vi "HFRR ADV v037.vi"() -> ()   [LabVIEW 2025] (continued)
                n805 = local write "EVENT LOG"(w838) -> ()
              }
            }
          }
        }
        n806 = case shown="True" w816 {
          frame False {
          }
          frame True {
            n807 = case shown="True" "Reach point temp" {
              selector: "Reach point temp" -> [_ w846]
              frame False {
              }
              frame True {
                n808 = local read "EVENT LOG"() -> (w843:string)
                n809 = Not(x=w846) -> (.not. x?=w845:bool)
                n810 = local write "Reach point temp"(w845) -> ()
                n811 = call "Event Log.vi"("Content"="Target Temperature reached", "EVENT LOG"=w843) -> ("EVENT LOG"=w844:string)  [unwired: 8 in, 1 out]
                n812 = local write "EVENT LOG"(w844) -> ()
              }
            }
          }
        }
        n813 = local read "Auto Start Test"() -> (w819:bool)
        n814 = And(x=w816, y=w815) -> (x .and. y?=w825:bool)
        n815 = Select(t=Auto_Start_enum."Maintain Stage" ("Enum - Selector"), s=w825, f=Auto_Start_enum."Reach point" ("Enum - Selector")) -> (s? t:f=w822:T15)
        n816 = Not(x=w819) -> (.not. x?=w818:bool)
        n817 = Select(t=Auto_Start_enum."close", s=w818, f=w822) -> (s? t:f=w820:T15)
        n818 = call "ELAPSED TIMER VI.vi"("RESET"=w821, "PAUSE"=w821) -> ()  [unwired: 7 in, 3 out]
      }
      frame "Maintain Stage" {
        w861 = 2.0 ("y")
        w860 = 1.0 ("y")
        # "Humidity and  temperatures Set Point  have been reached"
        n819 = local read "Set Temp"() -> (w847:dbl)
        n820 = local read "Set Humidity:"() -> (w864:dbl)
        n821 = local read "Humidity ( %RH )"() -> (w867:dbl)
        n822 = Add(x=w847, y=w860) -> (x+y=w866:dbl)
        n823 = Subtract(x=w847, y=w860) -> (x-y=w865:dbl)
        n824 = local read "TEMP"() -> (w868:dbl)
        n825 = Add(x=w864, y=w861) -> (x+y=w863:dbl)
        n826 = Subtract(x=w864, y=w861) -> (x-y=w862:dbl)
        n827 = In Range and Coerce(upper limit=w866, x=w868, lower limit=w865) -> (In Range?=w859:bool)  [unwired: 1 out]
        n828 = In Range and Coerce(upper limit=w863, x=w867, lower limit=w862) -> (In Range?=w858:bool)  [unwired: 1 out]
        n829 = And(x=w859, y=w858) -> (x .and. y?=w857:bool)
        n830 = Not(x=w857) -> (.not. x?=w856:bool)
        n831 = call "ELAPSED TIMER VI.vi"("TARGET"=60.0, "RESET"=w856, "PAUSE"=FALSE) -> ("ELAPSED INDICATION"=w853:bool)  [unwired: 6 in, 2 out]
        n832 = case shown="True" w853 {
          tunnel: w853 -> [_ w871]
          tunnel: [Auto_Start_enum."Maintain Stage" ("Enum - Selector") w870] -> w851
          frame False {
          }
          frame True {
            n833 = stacked-sequence {
              tunnel: w871 -> [_ _ _ _ _]
              tunnel: [_ _ _ _ Auto_Start_enum."Start Stage" ("Enum - Selector")] -> w870
              frame #0 {
                n834 = local read "EVENT LOG"() -> (w873:string)
                n835 = call "Event Log.vi"("Content"="Humidity and temperature set point has stabilized.", "EVENT LOG"=w873) -> ("EVENT LOG"=w874:string)  [unwired: 8 in, 1 out]
                n836 = local write "EVENT LOG"(w874) -> ()
              }
              frame #1 {
                n837 = Wait (ms)(milliseconds to wait=u32 100) -> ()  [unwired: 1 out]
              }
              frame #2 {
                n838 = local read "EVENT LOG"() -> (w877:string)
                n839 = call "Event Log.vi"("Content"="Auto Test Started", "EVENT LOG"=w877) -> ("EVENT LOG"=w878:string)  [unwired: 8 in, 1 out]
                n840 = local write "EVENT LOG"(w878) -> ()
              }
              frame #3 {
                w879 = TRUE ("RUN")
                n841 = local write "RUN"(w879) -> ()
                n842 = property on="Auto Start Temp" class="Bool (strict)"("Val(Sgnl)"=w879) -> ()  [unwired: 2 in, 2 out]
                "Auto Start Temp" <- w879
              }
              frame #4 {
              }
            }
          }
        }
        n843 = local read "Auto Start Test"() -> (w850:bool)
        n844 = Not(x=w850) -> (.not. x?=w849:bool)
        n845 = Select(t=Auto_Start_enum."close", s=w849, f=w851) -> (s? t:f=w852:T15)
      }
      frame "Start Stage" {
        w881 = TRUE ("PAUSE")
        n846 = local read "Auto Start Test"() -> (w886:bool)
        n847 = Not(x=w886) -> (.not. x?=w885:bool)
        n848 = Select(t=Auto_Start_enum."close" ("Enum - Selector"), s=w885, f=Auto_Start_enum."Start Stage" ("Enum - Selector")) -> (s? t:f=w882:T15)
        n849 = call "ELAPSED TIMER VI.vi"("RESET"=w881, "PAUSE"=w881) -> ()  [unwired: 7 in, 3 out]
      }
      frame "close" {
        w889 = FALSE ("Heater Button")
        n850 = local write "RUN"(w889) -> ()
        n851 = local write "Heater Button"(w889) -> ()
        n852 = local write "Humidity"(w889) -> ()
        n853 = local write "Auto Start Test"(w889) -> ()
        n854 = property on="Heater Button" class="Bool (strict)"("Val(Sgnl)"=FALSE ("Value (Signaling)")) -> ()  [unwired: 2 in, 2 out]
        n855 = local write "Humidity"(TRUE ("Humidity")) -> ()
      }
      frame "Exit" {
      }
    }
    n856 = Wait (ms)(milliseconds to wait=u32 100) -> ()  [unwired: 1 out]
    n857 = local read "Quit"() -> (w784:bool)
  }
  n858 = property on="Service Password Log" class="Str"("Visible"=w21) -> ()  [unwired: 2 in, 2 out]
  n859 = property on="Password 3" class="Clust (strict)"("Visible"=w21) -> ()  [unwired: 2 in, 2 out]
  n860 = while {
    stop <- w918 stop-if-true
    w901 = errorcluster {"status"=FALSE, "code"=0, "source"=""} ("error in (no error) 3")
    # "this loop is for manual report generation"
    n861 = local read "Confirm Measrurement"() -> (w900:bool)
    n862 = case shown="True" w900 {
      selector: w900 -> [_ w1008]
      tunnel: errorcluster {"status"=FALSE, "code"=0, "source"=""} ("error in (no error) 3") -> [_ w1009]
      tunnel: [_ w1007] -> _
      frame False {
      }
      frame True {
        n863 = stacked-sequence {
          tunnel: w1009 -> [_ w1042 _]
          tunnel: w1008 -> [_ _ w1149]
          tunnel: [_ w1030 _] -> w1007
          frame #0 {
            n864 = String To Path(string="C:\\LAB-IQ\\Image Calibrate v01.dcf") -> (path=w1012:path)
            n865 = Open/Create/Replace File ("Open File")(file path (use dialog)=w1012) -> (refnum out=w1013:refnum<file>)  [unwired: 5 in, 2 out]
            n866 = for {
              N: 4 -> [_]
              tunnel: w1013 -> [w1019]
              i -> [w1015]
              n867 = Read from Text File ("Read File")(file (use dialog)=w1019) -> (text=w1020:string)  [unwired: 3 in, 3 out]
              n868 = String Subset(string=w1020, offset (0)=6, length (rest)=10 ("length (rest)")) -> (substring=w1016:string)
              n869 = Fract/Exp String To Number(string=w1016) -> (number=w1014:dbl)  [unwired: 3 in, 1 out]
              n870 = case shown="3" w1015 {
                tunnel: w1014 -> [w1021 w1022 _ w1023 _]
                frame 0 {
                  n871 = local write "5x Gain"(w1021) -> ()
                }
                frame 1 {
                  n872 = local write "10x Gain"(w1022) -> ()
                }
                frame 2 {
                }
                frame 3 {
                  n873 = local write "100x gain"(w1023) -> ()
                }
                frame 4, Default {
                }
              }
            }
          }
          frame #1 {
            n874 = local read "TEST STANDARD"() -> (w1025:T3)
            n875 = case shown="\"ISO 12156\"" w1025 {
              tunnel: ["ASTM D6079" "ISO 12156"] -> w1024
              frame "ASTM D6079", Default {
              }
              frame "ISO 12156" {
              }
            }
            n876 = call "IMAGE ANALYSIS.vi"("Enum"=POST_ANALYSIS_ENUM."GET MEASUREMENTS", "error in"=w1042) -> ("error out"=w1049:errorcluster)  [unwired: 8 in, 1 out]
            n877 = local read "Magnification :"() -> (w1035:string)
            n878 = call "Stall Data Flow.vim"("value in"=w1049, "milliseconds to wait"=u32 1000) -> ("value out"=w1048:errorcluster)  [unwired: 1 out]
            n879 = local read "Test File List :"() -> (w1046:string)
            n880 = case shown="\"10x\"" w1035 {
              tunnel: [w1085 w1086] -> w1033
              frame "5x", Default {
                n881 = local read "5x Gain"() -> (w1085:dbl)
              }
              frame "10x" {
                # "5x"
                n882 = local read "10x Gain"() -> (w1086:dbl)
              }
            }
            n883 = call "IMAGE ANALYSIS.vi"("Enum"=POST_ANALYSIS_ENUM."READ", "error in"=w1048) -> ("error out"=w1045:errorcluster, "data out"=w1036:string)  [unwired: 8 in]
            n884 = Match Pattern(string=w1036, regular expression="\"type\": ") -> (after substring=w1040:string)  [unwired: 1 in, 3 out]
            n885 = call "IMAGE PATH CREATION PY.vi"("error in (no error)"=w1045, "File Name :"=w1046) -> ("error out"=w1044:errorcluster, "File Path"=w1032:path, "File Path String:"=w1027:string)  [unwired: 7 in]
            n886 = Match Pattern(string=w1040, regular expression=",") -> (before substring=w1026:string)  [unwired: 1 in, 3 out]
            n887 = local read "Calibration Tab"() -> (w1029:enum32{"Measrument", "Calibrate"})
            n888 = call "Stall Data Flow.vim"("value in"=w1044, "milliseconds to wait"=u32 250) -> ("value out"=w1028:errorcluster)  [unwired: 1 out]
            n889 = Equal?(x=w1026, y="\"rectangle\"") -> (x = y?=w1037:bool)
            n890 = case shown="False" w1037 {
              tunnel: w1036 -> [w1091 w1146]
              tunnel: w1033 -> [_ w1137]
              tunnel: cluster{"major":dbl, "minor":dbl, "average":dbl} {"major"=0.0, "minor"=0.0, "average"=0.0} -> [w1089 w1133]
              tunnel: [w1088 w1130] -> w1031
              tunnel: w1026 -> [w1090 _]
              tunnel: w1033 -> [w1087 _]
              frame False {
                n891 = Equal?(x=w1090, y="\"line\"") -> (x = y?=w1092:bool)
                n892 = case shown="True" w1092 {
                  tunnel: w1091 -> [_ w1107]
                  tunnel: w1089 -> [w1094 w1106]
                  tunnel: [w1094 w1104] -> w1088
                  tunnel: w1087 -> [_ w1103]
                  frame False {
                  }
                  frame True {
                    w1102 = 0.0 ("Major Axis")
                    n893 = Match Pattern(string=w1107, regular expression="\"length_px\":") -> (after substring=w1105:string)  [unwired: 1 in, 3 out]
                    n894 = property on="Major Axis" class="DigNum (strict)"("Caption.Text"="") -> ()  [unwired: 2 in, 2 out]
                    n895 = property on="Minor Axis" class="DigNum (strict)"("Caption.Text"="") -> ()  [unwired: 2 in, 2 out]
                    n896 = property on="Average" class="DigNum (strict)"("Caption.Text"="Line") -> ()  [unwired: 2 in, 2 out]
                    n897 = Fract/Exp String To Number(string=w1105, default (0 dbl)=0.0 ("default (0 DBL)")) -> (number=w1101:dbl)  [unwired: 2 in, 1 out]
                    "Pixel Value" <- w1101
                    n898 = Multiply(x=w1101, y=w1103) -> (x*y=w1114:dbl)
                    n899 = Multiply(x=w1114, y=1000.0) -> (x*y=w1097:dbl)
                    n900 = Divide(x=w1097, y=1000.0) -> (x/y=w1100:dbl)
                    n901 = local write "Measurment (mm)"(w1100) -> ()
                    n902 = Bundle By Name(cluster=w1106, "average"=w1097) -> (w1104:cluster{"major":dbl, "minor":dbl, "average":dbl})
                    n903 = Number To Fractional String(number=w1097, precision (6)=i16 1) -> (F-format string=w1096:string)  [unwired: 2 in]
                    n904 = local write "Minor Axis"(w1102) -> ()
                    n905 = local write "Major Axis"(w1102) -> ()
                    n906 = Fract/Exp String To Number(string=w1096) -> (number=w1095:dbl)  [unwired: 3 in, 1 out]
                    n907 = local write "Average"(w1095) -> ()
                  }
                }
              }
              frame True {
                w1134 = 1000.0 ("y")
                w1140 = 0.0 ("default (0 DBL)")
                n908 = Match Pattern(string=w1146, regular expression=" \"width_px\":") -> (after substring=w1144:string)  [unwired: 1 in, 3 out]
                n909 = Match Pattern(string=w1144, regular expression="\"height_px\":") -> (before substring=w1142:string, after substring=w1141:string)  [unwired: 1 in, 2 out]
                n910 = Fract/Exp String To Number(string=w1142, default (0 dbl)=w1140) -> (number=w1139:dbl)  [unwired: 2 in, 1 out]
                n911 = Fract/Exp String To Number(string=w1141, default (0 dbl)=w1140) -> (number=w1138:dbl)  [unwired: 2 in, 1 out]
                n912 = Multiply(x=w1139, y=w1137) -> (x*y=w1136:dbl)
                n913 = Multiply(x=w1138, y=w1137) -> (x*y=w1135:dbl)
                n914 = Multiply(x=w1136, y=w1134) -> (x*y=w1120:dbl)
                n915 = Multiply(x=w1135, y=w1134) -> (x*y=w1118:dbl)
                n916 = Add(x=w1120, y=w1118) -> (x+y=w1132:dbl)
                n917 = property on="Major Axis" class="DigNum (strict)"("Caption.Text"="Major Axis") -> ()  [unwired: 2 in, 2 out]
                n918 = property on="Minor Axis" class="DigNum (strict)"("Caption.Text"="Minor Axis") -> ()  [unwired: 2 in, 2 out]
                n919 = property on="Average" class="DigNum (strict)"("Caption.Text"="Average") -> ()  [unwired: 2 in, 2 out]
                n920 = Divide(x=w1132, y=2.0) -> (x/y=w1116:dbl)
                n921 = Bundle By Name(cluster=w1133, "major"=w1120, "minor"=w1118, "average"=w1116) -> (w1130:cluster{"major":dbl, "minor":dbl, "average":dbl})
                n922 = Number To Fractional String(number=w1118, precision (6)=i16 1) -> (F-format string=w1125:string)  [unwired: 2 in]
                n923 = Number To Fractional String(number=w1116, precision (6)=i16 1) -> (F-format string=w1126:string)  [unwired: 2 in]
                n924 = Number To Fractional String(number=w1120, precision (6)=i16 1) -> (F-format string=w1124:string)  [unwired: 2 in]
                n925 = Fract/Exp String To Number(string=w1125) -> (number=w1117:dbl)  [unwired: 3 in, 1 out]
                n926 = Fract/Exp String To Number(string=w1126) -> (number=w1115:dbl)  [unwired: 3 in, 1 out]
                n927 = Fract/Exp String To Number(string=w1124) -> (number=w1119:dbl)  [unwired: 3 in, 1 out]
                n928 = local write "Major Axis"(w1119) -> ()
                n929 = local write "Average"(w1115) -> ()
                n930 = local write "Minor Axis"(w1117) -> ()
              }
            }
            n931 = case shown="\"Measrument\", Default" w1029 {
              tunnel: w1032 -> [w1059 _]
              tunnel: w1031 -> [w1058 _]
              tunnel: [w1055 w1084] -> w1030
              tunnel: w1028 -> [w1057 w1084]
              tunnel: w1027 -> [w1056 _]
              tunnel: w1024 -> [w1054 _]
              frame "Measrument", Default {
                n932 = stacked-sequence {
                  tunnel: w1059 -> [w1077 _]
                  tunnel: w1058 -> [w1075 _]
                  tunnel: w1057 -> [w1073 _]
                  tunnel: w1056 -> [w1072 _]
                  tunnel: [w1067 _] -> w1055
                  tunnel: w1054 -> [w1060 _]
                  frame #0 {
                    n933 = call "IMAGE ANALYSIS.vi"("Enum"=POST_ANALYSIS_ENUM."SAVE IMAGE", "error in"=w1073, "IMAGE FILE PATH"=w1072) -> ("error out"=w1071:errorcluster)  [unwired: 7 in, 1 out]
                    n934 = call "Stall Data Flow.vim"("value in"=w1071, "milliseconds to wait"=u32 1000) -> ("value out"=w1062:errorcluster)  [unwired: 1 out]
                    n935 = local read "Test File List :"() -> (w1079:string)
                    n936 = call "IMAGE ANALYSIS.vi"("Enum"=POST_ANALYSIS_ENUM."MINIMIZE UI", "error in"=w1062) -> ("error out"=w1069:errorcluster)  [unwired: 8 in, 1 out]
                    n937 = Bundle By Name(cluster=T27 {"File Name"="", "Test Method"="", "Operator"="", "Fuel Description"="", "Date and time"=""} ("Main Ref"), "Test Method"=w1060, "File Name"=w1079) -> (w1080:T27)
                    n938 = call "Stall Data Flow.vim"("value in"=w1069, "milliseconds to wait"=u32 1500) -> ("value out"=w1064:errorcluster)  [unwired: 1 out]
                    n939 = call "duf file read.vi"("error in (no error)"=w1064, "Main Ref"=w1080) -> ("error out"=w1078:errorcluster, "Main Ref 2"=w1076:T27)  [unwired: 8 in]
                    n940 = call "DETECTION REPORT for manual.vi"("error in (no error)"=w1078, "return value 3"=w1075, "Image File Path"=w1077, "Main Ref"=w1076) -> ("error out"=w1074:errorcluster)  [unwired: 7 in]
                    n941 = call <vilib>:"Clear Errors.vi"("error in (no error)"=w1074) -> ("error out"=w1065:errorcluster)  [unwired: 5 in, 1 out]
                    n942 = call "IMAGE ANALYSIS.vi"("Enum"=POST_ANALYSIS_ENUM."MINIMIZE UI", "error in"=w1065) -> ("error out"=w1067:errorcluster)  [unwired: 8 in, 1 out]
                  }
                  frame #1 {
                    n943 = local write "Main Tab"(T2."HOME" ("Main Tab")) -> ()
                    n944 = local write "Main Dashboard Buttons"(T1."Home" ("Main Dashboard Buttons")) -> ()
                  }
                }
              }
              frame "Calibrate" {
              }
            }
          }
          frame #2 {
            n945 = Not(x=w1149) -> (.not. x?=w1148:bool)
            n946 = local write "Confirm Measrurement"(w1148) -> ()
            n947 = local read "Calibration Tab"() -> (w1147:enum32{"Measrument", "Calibrate"})
            n948 = case shown="\"Measrument\", Default" w1147 {
              frame "Measrument", Default {
                (unwired) T21."HOME" ("Main Tab")
                n949 = local write "Main Tab"(T2."HOME" ("Main Tab")) -> ()
              }
              frame "Calibrate" {
              }
            }
          }
        }
      }
    }
    n950 = local read "Humidity"() -> (w892:bool)
    n951 = local read "Save Change"() -> (w897:bool)
    n952 = local read "Calibrate"() -> (w898:bool)
    n953 = local read "Auto Start Test"() -> (w893:bool)
    n954 = case shown="True" w898 {
      selector: w898 -> [_ w1005]
      frame False {
      }
      frame True {
        n955 = Not(x=w1005) -> (.not. x?=w1004:bool)
        n956 = local write "Calibrate"(w1004) -> ()
        n957 = local write "Calibration Tab"(enum32{"Measrument", "Calibrate"}."Calibrate" ("Calibration Tab")) -> ()
      }
    }
    n958 = case shown="True" w897 {
      selector: w897 -> [_ w949]
      frame False {
      }
      frame True {
        n959 = stacked-sequence {
          tunnel: w949 -> [_ _ _ _ w1003]
          frame #0 {
            n960 = call "IMAGE ANALYSIS.vi"("Enum"=POST_ANALYSIS_ENUM."HIDE UI") -> ()  [unwired: 9 in, 2 out]
          }
          frame #1 {
            n961 = local read "100x gain"() -> (w951:dbl)
            n962 = local read "10x Gain"() -> (w952:dbl)
            n963 = local read "5x Gain"() -> (w953:dbl)
            n964 = Number To Fractional String(number=w952, width (-)=i16 4, precision (6)=i16 7) -> (F-format string=w974:string)  [unwired: 1 in]
            n965 = Number To Fractional String(number=0.0, width (-)=i16 4, precision (6)=i16 7) -> (F-format string=w969:string)  [unwired: 1 in]
            n966 = Number To Fractional String(number=w951, width (-)=i16 4, precision (6)=i16 7) -> (F-format string=w957:string)  [unwired: 1 in]
            n967 = Number To Fractional String(number=w953, width (-)=i16 10 ("precision (6)"), precision (6)=i16 7) -> (F-format string=w983:string)  [unwired: 1 in]
            n968 = Concatenate Strings("[CH1]" ("string"), w983, " - 5x Gain" ("string"), "\r") -> (w973:string)
            n969 = Concatenate Strings("[CH2]" ("string"), w974, " - 10x Gain" ("string"), "\r") -> (w972:string)
            n970 = Concatenate Strings("[CH3]" ("string"), w969, " - 20x Gain" ("string"), "\r") -> (w963:string)
            n971 = Concatenate Strings("[CH4]" ("string"), w957, " - 100x Gain" ("string"), "\r") -> (w956:string)
            n972 = String To Path(string="C:\\LAB-IQ\\Image Calibrate v01.dcf") -> (path=w986:path)
            n973 = Concatenate Strings(w973, w972, w963, w956) -> (w971:string)
            n974 = call <vilib>:"Write Characters To File.vi"("append to file? (new file:F)"=FALSE, "character string"=w971, "file path (dialog if empty)"=w986) -> ()  [unwired: 2 in, 1 out]
          }
          frame #2 {
            n975 = String To Path(string="C:\\LAB-IQ\\Image Calibrate v01.dcf") -> (path=w989:path)
            n976 = Open/Create/Replace File ("Open File")(file path (use dialog)=w989) -> (refnum out=w990:refnum<file>)  [unwired: 5 in, 2 out]
            n977 = for {
              N: 4 -> [_]
              tunnel: w990 -> [w996]
              i -> [w992]
              n978 = Read from Text File ("Read File")(file (use dialog)=w996) -> (text=w997:string)  [unwired: 3 in, 3 out]
              n979 = String Subset(string=w997, offset (0)=6, length (rest)=10 ("length (rest)")) -> (substring=w993:string)
              n980 = Fract/Exp String To Number(string=w993) -> (number=w991:dbl)  [unwired: 3 in, 1 out]
              n981 = case shown="3" w992 {
                tunnel: w991 -> [w998 w999 _ w1000 _]
                frame 0 {
                  n982 = local write "5x Gain"(w998) -> ()
                }
                frame 1 {
                  n983 = local write "10x Gain"(w999) -> ()
                }
                frame 2 {
                }
                frame 3 {
                  n984 = local write "100x gain"(w1000) -> ()
                }
                frame 4, Default {
                }
              }
            }
          }
          frame #3 {
            n985 = call "IMAGE ANALYSIS.vi"("Enum"=POST_ANALYSIS_ENUM."SHOW UI") -> ()  [unwired: 9 in, 2 out]
          }
          frame #4 {
            n986 = Not(x=w1003) -> (.not. x?=w1002:bool)
            n987 = local write "Save Change"(w1002) -> ()
          }
        }
      }
    }
    n988 = case shown="False" w893 {
      tunnel: w892 -> [w919 _]
      frame False {
        n989 = case shown="True" w919 {
          frame False {
          }
          frame True {
            n990 = local read "Set Humidity:"() -> (w923:dbl)
            n991 = local read "Set Humidity:"() -> (w926:dbl)
            n992 = local read "Humidity ( %RH )"() -> (w927:dbl)
            n993 = Subtract(x=w923, y=2.0) -> (x-y=w921:dbl)
            n994 = Add(x=w926, y=2.0) -> (x+y=w922:dbl)
            n995 = In Range and Coerce(upper limit=w922, x=w927, lower limit=w921) -> (In Range?=w920:bool)  [unwired: 1 out]
            n996 = case shown="True" w920 {
              frame False {
              }
              frame True {
                n997 = case shown="True" "Manual Humididty Reached" {
                  selector: "Manual Humididty Reached" -> [_ w930]
                  frame False {
                  }
                  frame True {
                    n998 = Not(x=w930) -> (.not. x?=w929:bool)
                    n999 = local write "Manual Humididty Reached"(w929) -> ()
                    n1000 = local read "EVENT LOG"() -> (w932:string)
                    n1001 = call "Event Log.vi"("Content"="Target Humidity reached", "EVENT LOG"=w932) -> ("EVENT LOG"=w931:string)  [unwired: 8 in, 1 out]
                    n1002 = local write "EVENT LOG"(w931) -> ()
                  }
                }
              }
            }
          }
        }
      }
      frame True {
        n1003 = local write "Manual Humididty Reached"(TRUE ("Manual Humididty Reached")) -> ()
      }
    }
    n1004 = local read "Cap Live Image"() -> (w913:bool)
    n1005 = local read "SCAR MEASURMENT"() -> (w916:enum32{"Auto Scar", "Manual Scar"})
    n1006 = Wait (ms)(milliseconds to wait=u32 250) -> ()  [unwired: 1 out]
    n1007 = Equal?(x=w916, y=enum32{"Auto Scar", "Manual Scar"}."Manual Scar" ("SCAR MEASURMENT")) -> (x = y?=w914:bool)
    n1008 = And(x=w914, y=w913) -> (x .and. y?=w912:bool)
    n1009 = case shown="True" w912 {
      selector: w912 -> [_ w1228]
      frame False {
      }
      frame True {
        n1010 = stacked-sequence {
          tunnel: [_ _ _ w1243 _] -> _
          tunnel: w1228 -> [_ _ _ _ w1250]
          frame #0 {
            w1229 = 0.0
            n1011 = local write "Major Axis"(w1229) -> ()
            n1012 = local write "Minor Axis"(w1229) -> ()
            n1013 = local write "Average"(w1229) -> ()
          }
          frame #1 {
            n1014 = call "CAMERA LIVE FEED FGV.vi"("Enum - Menu"=CAMERA_LIVE_FEED_ENUM."CAMERA MINIMIZE") -> ()  [unwired: 9 in, 2 out]
          }
          frame #2 {
            n1015 = local read "FILE 3"() -> (w1237:string)
            n1016 = call <vilib>:"Trim Whitespace.vi"("string"="C:\\LAB-IQ\\images\\") -> ("trimmed string"=w1239:string)  [unwired: 1 in]
            n1017 = String To Path(string=w1239) -> (path=w1238:path)
            n1018 = Concatenate Strings(w1237, ".png" ("string")) -> (w1236:string)
            n1019 = Build Path(base path=w1238, name or relative path=w1236) -> (appended path=w1234:path)
            n1020 = Path To String(path=w1234) -> (string=w1233:string)
            n1021 = call "CAMERA LIVE FEED FGV.vi"("Enum - Menu"=CAMERA_LIVE_FEED_ENUM."CAMERA SAVE", "Image Path"=w1233) -> ("error out"=w1231:errorcluster)  [unwired: 8 in, 1 out]
            n1022 = case shown="No Error" w1231 {
              frame No Error {
                n1023 = One Button Dialog(message="Image saved successfully") -> ()  [unwired: 1 in, 1 out]
              }
              frame Error {
              }
            }
          }
          frame #3 {
            n1024 = call "LIST FILE NAMES.vi"() -> ("error out"=w1245:errorcluster, "filenames"=w1242:string[])  [unwired: 10 in]
            n1025 = call "IMAGE ANALYSIS.vi"("Enum"=POST_ANALYSIS_ENUM."SHOW UI", "error in"=w1245) -> ("error out"=w1243:errorcluster)  [unwired: 8 in, 1 out]
            n1026 = property on="Test File List :" class="CmbBox"("Strings[]"=w1242) -> ()  [unwired: 2 in, 2 out]
          }
          frame #4 {
            (unwired) T26."Report" ("Main Dashboard Buttons")
            (unwired) T28."Report" ("Main Dashboard Buttons")
            n1027 = Not(x=w1250) -> (.not. x?=w1249:bool)
            n1028 = local write "Zoom Factore"(0.0 ("Zoom Factore")) -> ()
            n1029 = local write "Cap Live Image"(w1249) -> ()
            n1030 = local write "Main Tab"(T2."Adv Scar Report" ("Main Tab")) -> ()
            n1031 = property on="Cap Live Image" class="Bool (strict)"("BoolText.Text"="Capture Image" ("Boolean Text.Text")) -> ()  [unwired: 2 in, 2 out]
            n1032 = local write "Main Dashboard Buttons"(T1."Report" ("Main Dashboard Buttons")) -> ()
          }
        }
      }
    }
    n1033 = local read "change Gain"() -> (w896:bool)
    n1034 = local read "Back Square"() -> (w895:bool)
    n1035 = case shown="True" w896 {
      selector: w896 -> [_ w940]
      frame False {
      }
      frame True {
        n1036 = stacked-sequence {
          tunnel: w940 -> [_ w948]
          frame #0 {
            n1037 = local read "Actual (µm)"() -> (w944:dbl)
            n1038 = local read "Pixel Value"() -> (w943:dbl)
            n1039 = local read "Magnification :"() -> (w942:string)
            n1040 = Divide(x=w944, y=w943) -> (x/y=w941:dbl)
            n1041 = case shown="\"10x\"" w942 {
              tunnel: w941 -> [w945 w946]
              frame "10x" {
                n1042 = local write "10x Gain"(w945) -> ()
              }
              frame "5x", Default {
                n1043 = local write "5x Gain"(w946) -> ()
              }
            }
          }
          frame #1 {
            n1044 = Not(x=w948) -> (.not. x?=w947:bool)
            n1045 = local write "change Gain"(w947) -> ()
          }
        }
      }
    }
    n1046 = case shown="True" w895 {
      selector: w895 -> [_ w938]
      frame False {
      }
      frame True {
        n1047 = Not(x=w938) -> (.not. x?=w937:bool)
        n1048 = local write "Back Square"(w937) -> ()
        n1049 = local write "Calibration Tab"(enum32{"Measrument", "Calibrate"}."Measrument" ("Calibration Tab")) -> ()
      }
    }
    n1050 = local read "Rectangle Tool"() -> (w907:bool)
    n1051 = local read "Clear ROI Tool"() -> (w906:bool)
    n1052 = local read "Open Image"() -> (w911:bool)
    n1053 = local read "line tool"() -> (w908:bool)
    n1054 = local read "OUT"() -> (w909:bool)
    n1055 = local read "In"() -> (w910:bool)
    n1056 = case shown="True" w911 {
      selector: w911 -> [_ w1216]
      tunnel: [w1212 w1218] -> _
      tunnel: w901 -> [w1212 w1217]
      frame False {
      }
      frame True {
        n1057 = Not(x=w1216) -> (.not. x?=w1215:bool)
        n1058 = local write "Open Image"(w1215) -> ()
        n1059 = call "IMAGE ANALYSIS.vi"("Enum"=POST_ANALYSIS_ENUM."HIDE UI", "error in"=w1217) -> ("error out"=w1225:errorcluster)  [unwired: 8 in, 1 out]
        n1060 = call "File Dialog"("start path"=path "C:/LAB-IQ/images", "error in"=w1225) -> ("selected path"=w1214:path, "error out"=w1223:errorcluster)  [unwired: 10 in, 2 out]
        "Image path  2" <- w1214
        n1061 = call <vilib>:"Clear Errors.vi"("error in (no error)"=w1223) -> ("error out"=w1222:errorcluster)  [unwired: 5 in, 1 out]
        n1062 = call "IMAGE ANALYSIS.vi"("Enum"=POST_ANALYSIS_ENUM."OPEN FILE", "error in"=w1222, "File Path"=w1214) -> ("error out"=w1221:errorcluster)  [unwired: 7 in, 1 out]
        n1063 = call <vilib>:"Clear Errors.vi"("error in (no error)"=w1221) -> ("error out"=w1220:errorcluster)  [unwired: 5 in, 1 out]
        n1064 = call "IMAGE ANALYSIS.vi"("Enum"=POST_ANALYSIS_ENUM."SHOW UI", "error in"=w1220) -> ("error out"=w1218:errorcluster)  [unwired: 8 in, 1 out]
        n1065 = local write "Zoom Factore"(100.0 ("Zoom Factore")) -> ()
      }
    }
    n1066 = case shown="True" w909 {
      selector: w909 -> [_ w1197]
      tunnel: w901 -> [w1194 w1202]
      tunnel: [w1194 w1196] -> _
      frame False {
      }
      frame True {
        n1067 = Not(x=w1197) -> (.not. x?=w1195:bool)
        n1068 = local read "Zoom Factore"() -> (w1200:dbl)
        n1069 = local write "OUT"(w1195) -> ()
        n1070 = call "IMAGE ANALYSIS.vi"("Enum"=POST_ANALYSIS_ENUM."ZOOM OUT", "error in"=w1202) -> ("error out"=w1196:errorcluster)  [unwired: 8 in, 1 out]
        n1071 = Divide(x=w1200, y=1.2) -> (x/y=w1198:dbl)
        n1072 = local write "Zoom Factore"(w1198) -> ()
      }
    }
    n1073 = case shown="True" w910 {
      selector: w910 -> [_ w1206]
      tunnel: w901 -> [w1203 w1211]
      tunnel: [w1203 w1204] -> _
      frame False {
      }
      frame True {
        n1074 = Not(x=w1206) -> (.not. x?=w1205:bool)
        n1075 = local read "Zoom Factore"() -> (w1209:dbl)
        n1076 = local write "In"(w1205) -> ()
        n1077 = call "IMAGE ANALYSIS.vi"("Enum"=POST_ANALYSIS_ENUM."ZOOM IN", "error in"=w1211) -> ("error out"=w1204:errorcluster)  [unwired: 8 in, 1 out]
        n1078 = Multiply(x=w1209, y=1.2) -> (x*y=w1207:dbl)
        n1079 = local write "Zoom Factore"(w1207) -> ()
      }
    }
    n1080 = case shown="True" w906 {
      selector: w906 -> [_ w1178]
      tunnel: w901 -> [w1176 w1180]
      tunnel: [w1176 w1179] -> _
      frame False {
      }
      frame True {
        n1081 = Not(x=w1178) -> (.not. x?=w1177:bool)
        n1082 = local write "Clear ROI Tool"(w1177) -> ()
        n1083 = call "IMAGE ANALYSIS.vi"("Enum"=POST_ANALYSIS_ENUM."CLEAR ROI", "error in"=w1180) -> ("error out"=w1179:errorcluster)  [unwired: 8 in, 1 out]
      }
    }
    n1084 = case shown="True" w908 {
      selector: w908 -> [_ w1190]
      tunnel: w901 -> [w1188 w1193]
      tunnel: [w1188 w1191] -> _
      frame False {
      }
      frame True {
        n1085 = Not(x=w1190) -> (.not. x?=w1189:bool)
        n1086 = local write "line tool"(w1189) -> ()
        n1087 = call "IMAGE ANALYSIS.vi"("Enum"=POST_ANALYSIS_ENUM."DRAW LINE", "error in"=w1193) -> ("error out"=w1191:errorcluster)  [unwired: 8 in, 1 out]
      }
    }
    n1088 = case shown="True" w907 {
      selector: w907 -> [_ w1184]
      tunnel: w901 -> [w1182 w1186]
      tunnel: [w1182 w1185] -> _
      frame False {
      }
      frame True {
        n1089 = Not(x=w1184) -> (.not. x?=w1183:bool)
        n1090 = local write "Rectangle Tool"(w1183) -> ()
        n1091 = call "IMAGE ANALYSIS.vi"("Enum"=POST_ANALYSIS_ENUM."DRAW REC", "error in"=w1186) -> ("error out"=w1185:errorcluster)  [unwired: 8 in, 1 out]
      }
    }
    n1092 = local read "SCAR MEASURMENT"() -> (w894:enum32{"Auto Scar", "Manual Scar"})
    n1093 = local read "Fit to Screen Tool"() -> (w903:bool)
    n1094 = local read "Resize Tool"() -> (w902:bool)
    n1095 = case shown="\"Manual Scar\", Default" w894 {
      frame "Auto Scar" {
        n1096 = property on="Cap Live Image" class="Bool (strict)"("BoolText.Text"="Report" ("Boolean Text.Text")) -> ()  [unwired: 2 in, 2 out]
      }
      frame "Manual Scar", Default {
        n1097 = property on="Cap Live Image" class="Bool (strict)"("BoolText.Text"="Save Image" ("Boolean Text.Text")) -> ()  [unwired: 2 in, 2 out]
      }
    }
    n1098 = local read "ROI Color Tool"() -> (w904:bool)
    n1099 = local read "Pan Tool"() -> (w905:bool)
    n1100 = case shown="True" w905 {
      selector: w905 -> [_ w1172]
      tunnel: w901 -> [w1170 w1174]
      tunnel: [w1170 w1173] -> _
      frame False {
      }
      frame True {
        n1101 = Not(x=w1172) -> (.not. x?=w1171:bool)
        n1102 = call "IMAGE ANALYSIS.vi"("Enum"=POST_ANALYSIS_ENUM."PAN", "error in"=w1174) -> ("error out"=w1173:errorcluster)  [unwired: 8 in, 1 out]
        n1103 = local write "Pan Tool"(w1171) -> ()
      }
    }
    n1104 = case shown="True" w902 {
      selector: w902 -> [_ w1156]
      tunnel: w901 -> [w1151 w1153]
      tunnel: [w1151 w1152] -> _
      frame False {
      }
      frame True {
        n1105 = Not(x=w1156) -> (.not. x?=w1155:bool)
        n1106 = local write "Resize Tool"(w1155) -> ()
        n1107 = call "IMAGE ANALYSIS.vi"("Enum"=POST_ANALYSIS_ENUM."RESIZE MODE", "error in"=w1153) -> ("error out"=w1152:errorcluster)  [unwired: 8 in, 1 out]
      }
    }
    n1108 = case shown="True" w903 {
      selector: w903 -> [_ w1161]
      tunnel: [w1157 w1162] -> _
      tunnel: w901 -> [w1157 w1160]
      frame False {
      }
      frame True {
        n1109 = Not(x=w1161) -> (.not. x?=w1159:bool)
        n1110 = local write "Zoom Factore"(100.0 ("Zoom Factore")) -> ()
        n1111 = local write "Fit to Screen Tool"(w1159) -> ()
        n1112 = call "IMAGE ANALYSIS.vi"("Enum"=POST_ANALYSIS_ENUM."FIT", "error in"=w1160) -> ("error out"=w1162:errorcluster)  [unwired: 8 in, 1 out]
      }
    }
    n1113 = case shown="True" w904 {
      selector: w904 -> [_ w1167]
      tunnel: [w1164 w1168] -> _
      tunnel: w901 -> [w1164 w1165]
      frame False {
      }
      frame True {
        n1114 = Not(x=w1167) -> (.not. x?=w1166:bool)
        n1115 = local write "ROI Color Tool"(w1166) -> ()
        n1116 = call "IMAGE ANALYSIS.vi"("Enum"=POST_ANALYSIS_ENUM."SET ROI COLOR", "error in"=w1165) -> ("error out"=w1168:errorcluster)  [unwired: 8 in, 1 out]
      }
    }
    n1117 = local read "Quit"() -> (w918:bool)
  }
  n1118 = while {
    stop <- w1252 stop-if-true
    n1119 = local read "Image Path"() -> (w1255:path)
    n1120 = local read "Print 3"() -> (w1258:bool)
    n1121 = Equal?(x=w1255, y=path "") -> (x = y?=w1254:bool)
    n1122 = Not(x=w1254) -> (.not. x?=w1253:bool)
    n1123 = property on="Print 3" class="Bool (strict)"("Visible"=w1253) -> ()  [unwired: 2 in, 2 out]
    n1124 = case shown="True" w1258 {
      frame False {
        n1125 = local write "Rd"(TRUE ("Boolean 7")) -> ()
      }
      frame True {
        n1126 = flat-sequence {
          tunnel: [w1298] -> w1266
          tunnel: [w1285] -> w1264
          tunnel: [w1295] -> w1260
          tunnel: w1266 -> [w1307]
          tunnel: [w1307] -> w1265
          tunnel: w1264 -> [w1306]
          tunnel: [w1306] -> w1263
          tunnel: [w1304] -> w1262
          tunnel: [w1303] -> w1261
          tunnel: w1260 -> [w1303]
          tunnel: w1265 -> [w1309]
          tunnel: w1263 -> [w1310]
          tunnel: w1262 -> [_]
          tunnel: w1261 -> [w1308]
          frame #0 {
            n1127 = case shown="True" "Rd" {
              frame False {
              }
              frame True {
                n1128 = while {
                  tunnel: "abcdefABCDEF" ("string 2") -> [w1277]
                  shift-right: [w1275] -> w1269
                  shift-left: "" -> [w1274]
                  i -> [w1284]
                  stop <- w1283 stop-if-true
                  n1129 = Random Number (0-1)() -> (number: 0 to 1=w1278:dbl)
                  n1130 = Multiply(x=w1278, y=62.0) -> (x*y=w1280:dbl)
                  n1131 = Decrement(x="Length 2") -> (x-1=w1273:i16)
                  n1132 = To Word Integer(number=w1280) -> (16bit integer=w1281:i16)
                  n1133 = String Subset(string=w1277, offset (0)=w1281, length (rest)=1 ("length (rest)")) -> (substring=w1276:string)
                  n1134 = Greater Or Equal?(x=w1284, y=w1273) -> (x >= y?=w1283:bool)
                  n1135 = Concatenate Strings(w1276, w1274) -> (w1275:string)
                }
                "String 10" <- w1269
                n1136 = local write "Rd"(FALSE ("Boolean 7")) -> ()
              }
            }
          }
          frame #1 {
            w1296 = "_resized.jpg" ("command line")
            (unwired) ".jpg -resize 320x240 " ("string")
            (unwired) "Choose an Image File" ("prompt")
            # "-resize 1798x425"
            n1137 = local read "Image Path"() -> (w1290:path)
            n1138 = Strip Path(path=w1290) -> (stripped path=w1285:path, name=w1286:string)
            n1139 = Match Pattern(string=w1286, regular expression=".jpg") -> (before substring=→"before substring 2":string, after substring=→"after substring":string)  [unwired: 1 in, 2 out]
            n1140 = Match Pattern(string=w1286, regular expression="\\") -> (before substring=w1292:string)  [unwired: 1 in, 3 out]
            n1141 = Match Pattern(string=w1292, regular expression=".jpg") -> (before substring=w1291:string)  [unwired: 1 in, 3 out]
            n1142 = Concatenate Strings("cmd /c convert " ("string"), w1291, ".jpg -resize 320x240  " ("command line"), w1291, w1296) -> (w1299:string)
            n1143 = call <vilib>:"System Exec.vi"("run minimized? (F)"=TRUE, "wait until completion? (T)"=TRUE, "working directory"=w1285, "command line"=w1299) -> ("error out"=w1298:errorcluster)  [unwired: 4 in, 3 out]
            "error out 2" <- w1298
            n1144 = Concatenate Strings(w1291, w1296) -> (w1295:string)
          }
          frame #2 {
            n1145 = Wait (ms)(milliseconds to wait=u32 2000 ("millisecond timer value")) -> (millisecond timer value=w1304:u32)
          }
          frame #3 {
            n1146 = case shown="No Error" w1309 {
              tunnel: w1310 -> [w1313 _]
              tunnel: w1308 -> [w1311 _]
              frame No Error {
                (unwired) ".jpg" ("string")
                n1147 = Path To String(path=w1313) -> (string=w1317:string)
                n1148 = Concatenate Strings(w1317, "\\" ("string"), w1311) -> (w1316:string)
                n1149 = String To Path(string=w1316) -> (path=w1315:path)
                n1150 = call <vilib>:"Read JPEG File.vi"("path to JPEG file"=w1315) -> ("image data"=w1319:T16)  [unwired: 8 in, 2 out]
                "image data" <- w1319
                n1151 = local write "Print 3"(FALSE ("Print 2")) -> ()
                n1152 = call <vilib>:"Draw Flattened Pixmap.vi"("image data"=w1319) -> ("new picture"=→"new picture":picture)  [unwired: 8 in]
              }
              frame Error {
              }
            }
          }
        }
      }
    }
    n1153 = Wait (ms)(milliseconds to wait=u32 20 ("millisecond timer value")) -> ()  [unwired: 1 out]
    n1154 = local read "Quit"() -> (w1252:bool)
  }
  n1155 = while {
    tunnel: w38 -> [_]
    tunnel: w24 -> [_]
    stop <- w1349 stop-if-true
    # "New Adv Logics"
    n1156 = local read "Main Tab"() -> (w1330:T2)
    n1157 = local read "Main Tab"() -> (w1347:T2)
    n1158 = local read "Sign In"() -> (w1346:bool)
    n1159 = case shown="\"Adv Scar\"" w1330 {
      frame "HOME", Default {
        n1160 = local read "LIVE FEED MIN TEMP"() -> (w1482:bool)
        n1161 = local write "LIVE FEED MAX TEMP"(TRUE ("LIVE FEED MAX TEMP")) -> ()
        n1162 = local read "CAMERA ROI MIN TEMP"() -> (w1480:bool)
        n1163 = case shown="True" w1482 {
          selector: w1482 -> [_ w1489]
          frame False {
          }
          frame True {
            n1164 = Not(x=w1489) -> (.not. x?=w1488:bool)
            n1165 = local write "LIVE FEED MIN TEMP"(w1488) -> ()
            n1166 = call "CAMERA LIVE FEED FGV.vi"("Enum - Menu"=CAMERA_LIVE_FEED_ENUM."CAMERA MINIMIZE") -> ()  [unwired: 9 in, 2 out]
          }
        }
        n1167 = case shown="True" w1480 {
          selector: w1480 -> [_ w1486]
          frame False {
          }
          frame True {
            n1168 = Not(x=w1486) -> (.not. x?=w1485:bool)
            n1169 = local write "CAMERA ROI MIN TEMP"(w1485) -> ()
            n1170 = call "IMAGE ANALYSIS.vi"("Enum"=POST_ANALYSIS_ENUM."MINIMIZE UI") -> ()  [unwired: 9 in, 2 out]
          }
        }
        n1171 = local write "CAMERA ROI MAX TEMP"(TRUE ("CAMERA ROI MAX TEMP")) -> ()
      }
      frame "Test Setup" {
        n1172 = local read "LIVE FEED MIN TEMP"() -> (w1492:bool)
        n1173 = local read "CAMERA ROI MIN TEMP"() -> (w1490:bool)
        n1174 = local write "LIVE FEED MAX TEMP"(TRUE ("LIVE FEED MAX TEMP")) -> ()
        n1175 = case shown="True" w1492 {
          selector: w1492 -> [_ w1499]
          frame False {
          }
          frame True {
            n1176 = Not(x=w1499) -> (.not. x?=w1498:bool)
            n1177 = local write "LIVE FEED MIN TEMP"(w1498) -> ()
            n1178 = call "CAMERA LIVE FEED FGV.vi"("Enum - Menu"=CAMERA_LIVE_FEED_ENUM."CAMERA MINIMIZE") -> ()  [unwired: 9 in, 2 out]
          }
        }
        n1179 = case shown="True" w1490 {
          selector: w1490 -> [_ w1496]
          frame False {
          }
          frame True {
            n1180 = Not(x=w1496) -> (.not. x?=w1495:bool)
            n1181 = local write "CAMERA ROI MIN TEMP"(w1495) -> ()
            n1182 = call "IMAGE ANALYSIS.vi"("Enum"=POST_ANALYSIS_ENUM."MINIMIZE UI") -> ()  [unwired: 9 in, 2 out]
          }
        }
        n1183 = local write "CAMERA ROI MAX TEMP"(TRUE ("CAMERA ROI MAX TEMP")) -> ()
      }
      frame "Acquire" {
        n1184 = local read "LIVE FEED MIN TEMP"() -> (w1502:bool)
        n1185 = local write "LIVE FEED MAX TEMP"(TRUE ("LIVE FEED MAX TEMP")) -> ()
        n1186 = local read "CAMERA ROI MIN TEMP"() -> (w1500:bool)
        n1187 = case shown="True" w1502 {
          selector: w1502 -> [_ w1509]
          frame False {
          }
          frame True {
            n1188 = Not(x=w1509) -> (.not. x?=w1508:bool)
            n1189 = local write "LIVE FEED MIN TEMP"(w1508) -> ()
            n1190 = call "CAMERA LIVE FEED FGV.vi"("Enum - Menu"=CAMERA_LIVE_FEED_ENUM."CAMERA MINIMIZE") -> ()  [unwired: 9 in, 2 out]
          }
        }
        n1191 = case shown="True" w1500 {
          selector: w1500 -> [_ w1506]
          frame False {
          }
          frame True {
            n1192 = Not(x=w1506) -> (.not. x?=w1505:bool)
            n1193 = local write "CAMERA ROI MIN TEMP"(w1505) -> ()
            n1194 = call "IMAGE ANALYSIS.vi"("Enum"=POST_ANALYSIS_ENUM."MINIMIZE UI") -> ()  [unwired: 9 in, 2 out]
          }
        }
        n1195 = local write "CAMERA ROI MAX TEMP"(TRUE ("CAMERA ROI MAX TEMP")) -> ()
      }
      frame "Adv Scar" {
        n1196 = local read "CAMERA ROI MIN TEMP"() -> (w1510:bool)
        n1197 = case shown="True" "LIVE FEED MAX TEMP" {
          selector: "LIVE FEED MAX TEMP" -> [_ w1531]
          frame False {
          }
          frame True {
            n1198 = Not(x=w1531) -> (.not. x?=w1530:bool)
            n1199 = local write "LIVE FEED MAX TEMP"(w1530) -> ()
            n1200 = call "CAMERA LIVE FEED FGV.vi"("Enum - Menu"=CAMERA_LIVE_FEED_ENUM."CAMERA RESTORE") -> ("error out"=w1521:errorcluster)  [unwired: 9 in, 1 out]
            n1201 = Type Cast(type=30, x=0) -> (*(type *) &x=w1525:i32)
            n1202 = Add(x=w1525, y=48) -> (x+y=w1526:i32)
            n1203 = call "CAMERA LIVE FEED FGV.vi"("Enum - Menu"=CAMERA_LIVE_FEED_ENUM."CAMERA MODE SET", "error in (no error)"=w1521, "CAMERA MODE"=w1526) -> ("error out"=w1518:errorcluster)  [unwired: 7 in, 1 out]
            n1204 = call "CAMERA LIVE FEED FGV.vi"("Enum - Menu"=CAMERA_LIVE_FEED_ENUM."CAMERA GRAY", "error in (no error)"=w1518) -> ("error out"=w1517:errorcluster)  [unwired: 8 in, 1 out]
            n1205 = call "LIST FILE NAMES.vi"("error in (no error)"=w1517) -> ("error out"=w1527:errorcluster, "filenames"=w1528:string[])  [unwired: 9 in]
            n1206 = property on="FILE 3" class="CmbBox"(error in=w1527, "Strings[]"=w1528) -> ()  [unwired: 1 in, 2 out]
          }
        }
        n1207 = case shown="True" w1510 {
          selector: w1510 -> [_ w1516]
          frame False {
          }
          frame True {
            n1208 = Not(x=w1516) -> (.not. x?=w1515:bool)
            n1209 = local write "CAMERA ROI MIN TEMP"(w1515) -> ()
            n1210 = call "IMAGE ANALYSIS.vi"("Enum"=POST_ANALYSIS_ENUM."MINIMIZE UI") -> ()  [unwired: 9 in, 2 out]
          }
        }
        n1211 = local write "CAMERA ROI MAX TEMP"(TRUE ("CAMERA ROI MAX TEMP")) -> ()
        "LIVE FEED MIN TEMP" <- TRUE ("LIVE FEED MIN TEMP")
      }
      frame "Adv Scar Report" {
        n1212 = local read "CAMERA ROI MAX TEMP"() -> (w1532:bool)
        n1213 = local read "LIVE FEED MIN TEMP"() -> (w1534:bool)
        n1214 = local write "LIVE FEED MAX TEMP"(TRUE ("LIVE FEED MAX TEMP")) -> ()
        n1215 = case shown="True" w1534 {
          selector: w1534 -> [_ w1543]
          frame False {
          }
          frame True {
            n1216 = Not(x=w1543) -> (.not. x?=w1542:bool)
            n1217 = local write "LIVE FEED MIN TEMP"(w1542) -> ()
            n1218 = call "CAMERA LIVE FEED FGV.vi"("Enum - Menu"=CAMERA_LIVE_FEED_ENUM."CAMERA MINIMIZE") -> ()  [unwired: 9 in, 2 out]
          }
        }
        n1219 = case shown="True" w1532 {
          selector: w1532 -> [_ w1540]
          frame False {
          }
          frame True {
            n1220 = Not(x=w1540) -> (.not. x?=w1538:bool)
            n1221 = local write "CAMERA ROI MAX TEMP"(w1538) -> ()
            n1222 = call "IMAGE ANALYSIS.vi"("Enum"=POST_ANALYSIS_ENUM."SHOW UI") -> ("error out"=w1537:errorcluster)  [unwired: 9 in, 1 out]
            n1223 = call "LIST FILE NAMES.vi"("error in (no error)"=w1537) -> ("filenames"=w1536:string[])  [unwired: 9 in, 1 out]
            n1224 = property on="Test File List :" class="CmbBox"("Strings[]"=w1536) -> ()  [unwired: 2 in, 2 out]
          }
        }
        n1225 = local write "CAMERA ROI MIN TEMP"(TRUE ("CAMERA ROI MIN TEMP")) -> ()
      }
      frame "Compare Files" {
        n1226 = local read "LIVE FEED MIN TEMP"() -> (w1546:bool)
        n1227 = local write "LIVE FEED MAX TEMP"(TRUE ("LIVE FEED MAX TEMP")) -> ()
        n1228 = local read "CAMERA ROI MIN TEMP"() -> (w1544:bool)
        n1229 = case shown="True" w1546 {
          selector: w1546 -> [_ w1553]
          frame False {
          }
          frame True {
            n1230 = Not(x=w1553) -> (.not. x?=w1552:bool)
            n1231 = local write "LIVE FEED MIN TEMP"(w1552) -> ()
            n1232 = call "CAMERA LIVE FEED FGV.vi"("Enum - Menu"=CAMERA_LIVE_FEED_ENUM."CAMERA MINIMIZE") -> ()  [unwired: 9 in, 2 out]
          }
        }
        n1233 = case shown="True" w1544 {
          selector: w1544 -> [_ w1550]
          frame False {
          }
          frame True {
            n1234 = Not(x=w1550) -> (.not. x?=w1549:bool)
            n1235 = local write "CAMERA ROI MIN TEMP"(w1549) -> ()
            n1236 = call "IMAGE ANALYSIS.vi"("Enum"=POST_ANALYSIS_ENUM."MINIMIZE UI") -> ()  [unwired: 9 in, 2 out]
          }
        }
        n1237 = local write "CAMERA ROI MAX TEMP"(TRUE ("CAMERA ROI MAX TEMP")) -> ()
      }
      frame "About" {
        n1238 = local read "LIVE FEED MIN TEMP"() -> (w1556:bool)
        n1239 = local write "LIVE FEED MAX TEMP"(TRUE ("LIVE FEED MAX TEMP")) -> ()
        n1240 = local read "CAMERA ROI MIN TEMP"() -> (w1555:bool)
        n1241 = case shown="True" w1556 {
          selector: w1556 -> [_ w1563]
          frame False {
          }
          frame True {
            n1242 = Not(x=w1563) -> (.not. x?=w1562:bool)
            n1243 = local write "LIVE FEED MIN TEMP"(w1562) -> ()
            n1244 = call "CAMERA LIVE FEED FGV.vi"("Enum - Menu"=CAMERA_LIVE_FEED_ENUM."CAMERA MINIMIZE") -> ()  [unwired: 9 in, 2 out]
          }
        }
        n1245 = case shown="True" w1555 {
          selector: w1555 -> [_ w1560]
          frame False {
          }
          frame True {
            n1246 = Not(x=w1560) -> (.not. x?=w1559:bool)
            n1247 = local write "CAMERA ROI MIN TEMP"(w1559) -> ()
            n1248 = call "IMAGE ANALYSIS.vi"("Enum"=POST_ANALYSIS_ENUM."MINIMIZE UI") -> ()  [unwired: 9 in, 2 out]
          }
        }
        n1249 = local write "CAMERA ROI MAX TEMP"(TRUE ("CAMERA ROI MIN TEMP")) -> ()
      }
      frame "Advance" {
        n1250 = local read "LIVE FEED MIN TEMP"() -> (w1566:bool)
        n1251 = local write "LIVE FEED MAX TEMP"(TRUE ("LIVE FEED MAX TEMP")) -> ()
        n1252 = local read "CAMERA ROI MIN TEMP"() -> (w1564:bool)
        n1253 = case shown="True" w1566 {
          selector: w1566 -> [_ w1573]
          frame False {
          }
          frame True {
            n1254 = Not(x=w1573) -> (.not. x?=w1572:bool)
            n1255 = local write "LIVE FEED MIN TEMP"(w1572) -> ()
            n1256 = call "CAMERA LIVE FEED FGV.vi"("Enum - Menu"=CAMERA_LIVE_FEED_ENUM."CAMERA MINIMIZE") -> ()  [unwired: 9 in, 2 out]
          }
        }
        n1257 = local write "CAMERA ROI MAX TEMP"(TRUE ("CAMERA ROI MAX TEMP")) -> ()
        n1258 = case shown="True" w1564 {
          selector: w1564 -> [_ w1570]
          frame False {
          }
          frame True {
            n1259 = Not(x=w1570) -> (.not. x?=w1569:bool)
            n1260 = local write "CAMERA ROI MIN TEMP"(w1569) -> ()
            n1261 = call "IMAGE ANALYSIS.vi"("Enum"=POST_ANALYSIS_ENUM."MINIMIZE UI") -> ()  [unwired: 9 in, 2 out]
          }
        }
      }
      frame "Mooha" {
        n1262 = local read "LIVE FEED MIN TEMP"() -> (w1576:bool)
        n1263 = local write "LIVE FEED MAX TEMP"(TRUE ("LIVE FEED MAX TEMP")) -> ()
        n1264 = local read "CAMERA ROI MIN TEMP"() -> (w1574:bool)
        n1265 = case shown="True" w1576 {
          selector: w1576 -> [_ w1583]
          frame False {
          }
          frame True {
            n1266 = Not(x=w1583) -> (.not. x?=w1582:bool)
            n1267 = local write "LIVE FEED MIN TEMP"(w1582) -> ()
            n1268 = call "CAMERA LIVE FEED FGV.vi"("Enum - Menu"=CAMERA_LIVE_FEED_ENUM."CAMERA MINIMIZE") -> ()  [unwired: 9 in, 2 out]
          }
        }
        n1269 = local write "CAMERA ROI MAX TEMP"(TRUE ("CAMERA ROI MAX TEMP")) -> ()
        n1270 = case shown="True" w1574 {
          selector: w1574 -> [_ w1580]
          frame False {
          }
          frame True {
            n1271 = Not(x=w1580) -> (.not. x?=w1579:bool)
            n1272 = local write "CAMERA ROI MIN TEMP"(w1579) -> ()
            n1273 = call "IMAGE ANALYSIS.vi"("Enum"=POST_ANALYSIS_ENUM."MINIMIZE UI") -> ()  [unwired: 9 in, 2 out]
          }
        }
      }
    }
    n1274 = local read "Auto Start Test"() -> (w1321:bool)
    n1275 = case shown="True" "sign in temp" {
      frame False {
      }
      frame True {
        w1356 = 1 ("y")
        n1276 = local read "USERNAME"() -> (w1362:string)
        n1277 = local read "USER ID"() -> (w1359:string)
        n1278 = call <vilib>:"Trim Whitespace.vi"("string"=w1362) -> ("trimmed string"=w1361:string)  [unwired: 1 in]
        n1279 = call <vilib>:"Trim Whitespace.vi"("string"=w1359) -> ("trimmed string"=w1360:string)  [unwired: 1 in]
        n1280 = String Length(string=w1361) -> (length=w1358:i32)
        n1281 = String Length(string=w1360) -> (length=w1357:i32)
        n1282 = Greater?(x=w1358, y=w1356) -> (0:w1355:bool)
        n1283 = Greater?(x=w1357, y=w1356) -> (0:w1354:bool)
        n1284 = And(x=w1355, y=w1354) -> (x .and. y?=w1353:bool)
        n1285 = case shown="True" w1353 {
          frame False {
            n1286 = property on="Sign In" class="Bool (strict)"("DisabledEnum"=T19."Disabled" ("Disabled")) -> ()  [unwired: 2 in, 2 out]
          }
          frame True {
            n1287 = property on="Sign In" class="Bool (strict)"("DisabledEnum"=T19."Enabled" ("Disabled")) -> ()  [unwired: 2 in, 2 out]
          }
        }
      }
    }
    n1288 = local read "Air Temperature"() -> (w1338:bool)
    n1289 = local read "Coefficient Of Friction"() -> (w1339:bool)
    n1290 = case shown="False" w1321 {
      frame False {
        n1291 = local read "Auto stop temp"() -> (w1350:bool)
        n1292 = case shown="True" w1350 {
          frame False {
          }
          frame True {
            n1293 = local write "Auto Start Temp"(FALSE ("Auto Start Temp")) -> ()
          }
        }
      }
      frame True {
        "Auto stop temp" <- TRUE ("Auto stop temp")
      }
    }
    n1294 = local read "Humidity"() -> (w1337:bool)
    n1295 = case shown="\"HOME\"" w1347 {
      frame "HOME" {
        n1296 = local write "main tab sub"(enum32{"Page 1", "Page 2"}."Page 1" ("main tab sub")) -> ()
      }
      frame Default {
        n1297 = local write "main tab sub"(enum32{"Page 1", "Page 2"}."Page 2" ("main tab sub")) -> ()
      }
    }
    n1298 = case shown="True" w1346 {
      selector: w1346 -> [_ w1698]
      frame False {
      }
      frame True {
        n1299 = Not(x=w1698) -> (.not. x?=w1697:bool)
        n1300 = local write "Sign In"(w1697) -> ()
        n1301 = local write "Main Dashboard Buttons"(T26."Test Setup" ("Main Dashboard Buttons")) -> ()
      }
    }
    n1302 = case shown="\"Numeric Display\", Default" "Num/Graph" {
      frame "Numeric Display", Default {
        n1303 = property on="Single/Multiple" class="RadioBtnsControl (strict)"("Visible"=FALSE) -> ()  [unwired: 2 in, 2 out]
        n1304 = property on="Single - Graph" class="Ring (strict)"("Visible"=FALSE) -> ()  [unwired: 2 in, 2 out]
        n1305 = local write "Main Tab Display"(T4."Dashboard 1" ("Main Tab Display")) -> ()
      }
      frame "Graph Display" {
        n1306 = property on="Single/Multiple" class="RadioBtnsControl (strict)"("Visible"=TRUE) -> ()  [unwired: 2 in, 2 out]
        n1307 = case shown="\"Multiple\"" "Single/Multiple" {
          frame "Single ", Default {
            n1308 = property on="Single - Graph" class="Ring (strict)"("Visible"=TRUE) -> ()  [unwired: 2 in, 2 out]
            n1309 = local write "Main Tab Display"(T4."Dashboard 3" ("Main Tab Display")) -> ()
          }
          frame "Multiple" {
            n1310 = property on="Single - Graph" class="Ring (strict)"("Visible"=FALSE) -> ()  [unwired: 2 in, 2 out]
            n1311 = local write "Main Tab Display"(T4."Dashboard 2" ("Main Tab Display")) -> ()
          }
        }
      }
    }
    n1312 = local read "Stroke"() -> (w1336:bool)
    n1313 = local read "USERNAME"() -> (w1341:string)
    n1314 = case shown="True" w1339 {
      selector: w1339 -> [_ w1623]
      frame False {
      }
      frame True {
        n1315 = Not(x=w1623) -> (.not. x?=w1622:bool)
        n1316 = local write "Coefficient Of Friction"(w1622) -> ()
        n1317 = local write "Tab Control 2"(T6."Coefficient Of Friction" ("Tab Control 2")) -> ()
      }
    }
    n1318 = case shown="True" w1338 {
      selector: w1338 -> [_ w1620]
      frame False {
      }
      frame True {
        n1319 = Not(x=w1620) -> (.not. x?=w1618:bool)
        n1320 = local write "Air Temperature"(w1618) -> ()
        n1321 = local write "Tab Control 2"(T6."Air Temperature" ("Tab Control 2")) -> ()
      }
    }
    n1322 = case shown="True" w1336 {
      selector: w1336 -> [_ w1614]
      frame False {
      }
      frame True {